vi "FlexMag - 23-03-2023.vi"() -> ()   [LabVIEW 2018] (continued)
            n880 = local read "CH3_CC_DI"() -> (w1149:bool)
            n881 = local read "Tp3_stop_cmnd"() -> (w1127:bool)
            n882 = local read "CH3_BG_BV_DI"() -> (w1124:bool)
            n883 = local read "CH3_TP_BV_DI"() -> (w1122:bool)
            n884 = Compound Arithmetic op=AND(w1091, w1092) -> (w1095:bool)
            n885 = Compound Arithmetic op=AND(w1093, w1094) -> (w1096:bool)
            n886 = local read "Tp3 speed gui"() -> (w1121:i32)
            n887 = local read "CH3_CC_DI"() -> (w1123:bool)
            n888 = local read "CH3_SoV_Ar_DI"() -> (w1141:bool)
            n889 = Or(x=w1095, y=w1096) -> (x .or. y?=w1086:bool)
            n890 = Not(x=w1149) -> (.not. x?=w1148:bool)
            n891 = Not(x=w1147) -> (.not. x?=w1146:bool)
            n892 = Not(x=w1145) -> (.not. x?=w1144:bool)
            n893 = local write "ch3 trnsbp right open safety"(w1086) -> ()
            n894 = Less Or Equal?(x=w1121, y=180) -> (x <= y?=w1119:bool)
            n895 = Not(x=w1124) -> (.not. x?=w1125:bool)
            n896 = Not(x=w1123) -> (.not. x?=w1126:bool)
            n897 = Not(x=w1122) -> (.not. x?=w1120:bool)
            n898 = Compound Arithmetic op=AND(w1148, w1146, w1144) -> (w1142:bool)
            n899 = Compound Arithmetic op=AND(w1127, w1125, w1126, w1120, w1119, w1117) -> (w1118:bool)
            n900 = local write "sov3 open safety"(w1142) -> ()
            n901 = Compound Arithmetic op=AND(w1142, w1141) -> (w1143:bool)
            n902 = local write "chvbv3 open safety"(w1118) -> ()
            n903 = local write "ch3 mfc set safety"(w1143) -> ()
          }
          frame True {
            w1166 = TRUE ("bgbv3 open safety")
            n904 = local write "bgbv3 open safety"(w1166) -> ()
            n905 = local write "cc3 open safety"(w1166) -> ()
            n906 = local write "tpbv3 open safety"(w1166) -> ()
            n907 = local write "mp3 stop safety"(w1166) -> ()
            n908 = local write "tp3 start safety"(w1166) -> ()
            n909 = local write "tpbv3 close safety"(w1166) -> ()
            n910 = local write "mp3 start safety"(w1166) -> ()
            n911 = local write "plvbv3 open safety"(w1166) -> ()
            n912 = local write "sov3 open safety"(w1166) -> ()
            n913 = local write "ch3 mfc set safety"(w1166) -> ()
            n914 = local write "chvbv3 open safety"(w1166) -> ()
            n915 = local write "ch3 trnsbp left open safety"(w1166) -> ()
            n916 = local write "ch3 trnsbp right open safety"(w1166) -> ()
          }
        }
        n917 = case shown="False" "CH4 safety cancel" {
          frame False {
            n918 = local read "CH4_CH_VBV_DI"() -> (w1069:bool)
            n919 = local read "CH4_PL_VBV_DI"() -> (w1030:bool)
            n920 = local read "CH4_PL_ATM_DI"() -> (w997:bool)
            n921 = local read "CH3_SoV_Ar_DI"() -> (w1066:bool)
            n922 = local read "CH4_CH_ATM_DI"() -> (w996:bool)
            n923 = local read "ch4 ch pg torr"() -> (w1072:dbl)
            n924 = local read "Tp4_stop_cmnd"() -> (w1002:bool)
            n925 = local read "CH4_TP_BV_DI"() -> (w1017:bool)
            n926 = local read "CH4_MP_DI"() -> (w1026:bool)
            n927 = local read "ch3_4 vacuum level"() -> (w1014:string)
            n928 = local read "ch4 ch pg torr"() -> (w1012:dbl)
            n929 = local read "ch4 ch pg torr"() -> (w1011:dbl)
            n930 = Not(x=w1030) -> (.not. x?=w1029:bool)
            n931 = Not(x=w1069) -> (.not. x?=w1068:bool)
            n932 = Less Or Equal?(x=w1072, y=0.09) -> (x <= y?=w1070:bool)
            n933 = Not(x=w1066) -> (.not. x?=w1067:bool)
            n934 = Not(x=w1017) -> (.not. x?=w1018:bool)
            n935 = Compound Arithmetic op=XOR(w997, w996) -> (w999:bool)
            n936 = Compound Arithmetic op=AND(w1026, w1068, w1070) -> (w1065:bool)
            n937 = Not(x=w999) -> (.not. x?=w998:bool)
            n938 = Compound Arithmetic op=AND(w1018, w1002) -> (w1019:bool)
            n939 = Greater Or Equal?(x=w1012, y=0.9) -> (x >= y?=w1010:bool)
            n940 = Equal?(x="ATMOSPHERE" ("y"), y=w1014) -> (x = y?=w1009:bool)
            n941 = Equal?(x=w1014, y="VACUUM") -> (x = y?=w1007:bool)
            n942 = Less Or Equal?(x=w1011, y=0.1) -> (x <= y?=w1006:bool)
            n943 = Compound Arithmetic op=AND(w1065, w1067) -> (w1064:bool)
            n944 = local write "bgbv4 open safety"(w1065) -> ()
            n945 = Compound Arithmetic op=AND(w998, w1029) -> (w1031:bool)
            n946 = local write "mp4 stop safety"(w1019) -> ()
            n947 = local write "cc4 open safety"(w1064) -> ()
            n948 = Compound Arithmetic op=AND(w1010, w1009) -> (w1005:bool)
            n949 = Compound Arithmetic op=AND(w1007, w1006) -> (w1004:bool)
            n950 = local write "tpbv4 open safety"(w1031) -> ()
            n951 = Or(x=w1005, y=w1004) -> (x .or. y?=w1003:bool)
            n952 = local write "ch4 trnsbp right open safety"(w1003) -> ()
            n953 = local read "CH4_CH_VBV_DI"() -> (w1062:bool)
            n954 = local read "Tp4_stop_cmnd"() -> (w1027:bool)
            n955 = local read "CH4_TP_BV_DI"() -> (w1058:bool)
            n956 = local read "ch4 ch pg torr"() -> (w1059:dbl)
            n957 = local read "CH4_TP_BV_DI"() -> (w1045:bool)
            n958 = local read "CH4_CH_VBV_DI"() -> (w1023:bool)
            n959 = local read "CH4_MP_DI"() -> (w1057:bool)
            n960 = local read "CH4_PL_VBV_DI"() -> (w1024:bool)
            n961 = local read "ch4_tp_gui"() -> (w1001:bool)
            n962 = local read "CH4_MP_DI"() -> (w1046:bool)
            n963 = Not(x=w1062) -> (.not. x?=w1063:bool)
            n964 = Less Or Equal?(x=w1059, y=0.7) -> (x <= y?=w1061:bool)
            n965 = Not(x=w1001) -> (.not. x?=w1000:bool)
            n966 = Not(x=w1045) -> (.not. x?=w1044:bool)
            n967 = Not(x=w1046) -> (.not. x?=w1043:bool)
            n968 = Not(x=w1023) -> (.not. x?=w1021:bool)
            n969 = Not(x=w1024) -> (.not. x?=w1022:bool)
            n970 = Compound Arithmetic op=AND(w1063, w1061, w1058, w1057) -> (w1056:bool)
            n971 = Compound Arithmetic op=AND(w1000, w1027) -> (w1028:bool)
            n972 = Compound Arithmetic op=AND(w1044, w1043) -> (w1042:bool)
            n973 = Compound Arithmetic op=AND(w1022, w1021) -> (w1020:bool)
            n974 = local write "tp4 start safety"(w1056) -> ()
            n975 = local write "tpbv4 close safety"(w1028) -> ()
            n976 = local write "mp4 start safety"(w1020) -> ()
            n977 = local write "plvbv4 open safety"(w1042) -> ()
            n978 = local read "CH4_CH_ATM_DI"() -> (w1054:bool)
            n979 = local read "CH4_CH_VBV_DI"() -> (w1052:bool)
            n980 = local read "Tp4_stop_cmnd"() -> (w1025:bool)
            n981 = local read "CH4_BG_BV_DI"() -> (w1039:bool)
            n982 = local read "CH4_TP_BV_DI"() -> (w1037:bool)
            n983 = local read "CH4_CC_DI"() -> (w1050:bool)
            n984 = local read "Tp4 speed gui"() -> (w1036:i32)
            n985 = local read "CH4_CC_DI"() -> (w1038:bool)
            n986 = local read "CH4_SoV_Ar_DI"() -> (w1048:bool)
            n987 = Not(x=w1050) -> (.not. x?=w1051:bool)
            n988 = Not(x=w1052) -> (.not. x?=w1053:bool)
            n989 = Not(x=w1054) -> (.not. x?=w1055:bool)
            n990 = Less Or Equal?(x=w1036, y=180) -> (x <= y?=w1033:bool)
            n991 = Not(x=w1039) -> (.not. x?=w1040:bool)
            n992 = Not(x=w1038) -> (.not. x?=w1041:bool)
            n993 = Not(x=w1037) -> (.not. x?=w1034:bool)
            n994 = Compound Arithmetic op=AND(w1025, w1040, w1041, w1034, w1033) -> (w1032:bool)
            n995 = Compound Arithmetic op=AND(w1051, w1053, w1055) -> (w1047:bool)
            n996 = Compound Arithmetic op=AND(w1047, w1048) -> (w1049:bool)
            n997 = local write "sov4 open safety"(w1047) -> ()
            n998 = local write "chvbv4 open safety"(w1032) -> ()
            n999 = local write "ch4 mfc set safety"(w1049) -> ()
          }
          frame True {
            w1073 = TRUE ("bgbv3 open safety")
            n1000 = local write "bgbv4 open safety"(w1073) -> ()
            n1001 = local write "cc4 open safety"(w1073) -> ()
            n1002 = local write "tpbv4 open safety"(w1073) -> ()
            n1003 = local write "mp4 stop safety"(w1073) -> ()
            n1004 = local write "tp4 start safety"(w1073) -> ()
            n1005 = local write "tpbv4 close safety"(w1073) -> ()
            n1006 = local write "mp4 start safety"(w1073) -> ()
            n1007 = local write "plvbv4 open safety"(w1073) -> ()
            n1008 = local write "sov4 open safety"(w1073) -> ()
            n1009 = local write "ch4 mfc set safety"(w1073) -> ()
            n1010 = local write "chvbv4 open safety"(w1073) -> ()
            n1011 = local write "ch4 trnsbp right open safety"(w1073) -> ()
          }
        }
        n1012 = case shown="False" "coating safety cancel" {
          frame False {
            n1013 = local read "ch2 argon mfc actual"() -> (w941:dbl)
            n1014 = local read "ch3 argon mfc actual"() -> (w944:dbl)
            n1015 = local read "CH2_SoV_Ar_DI"() -> (w946:bool)
            n1016 = local read "CH3_SoV_Ar_DI"() -> (w945:bool)
            n1017 = local read "DCPS_ SW1 DI"() -> (w952:bool)
            n1018 = local read "DCPS_ SW2 DI"() -> (w950:bool)
            n1019 = local read "CH2_WFC_DI"() -> (w951:bool)
            n1020 = local read "CH3_WFC_DI"() -> (w949:bool)
            n1021 = Greater Or Equal?(x=w941, y=3.0) -> (x >= y?=w940:bool)
            n1022 = Greater Or Equal?(x=w944, y=3.0) -> (x >= y?=w939:bool)
            n1023 = Compound Arithmetic op=AND(w940, w946, w952, w951) -> (w948:bool)
            n1024 = Compound Arithmetic op=AND(w949, w950, w945, w939) -> (w947:bool)
            n1025 = Or(x=w948, y=w947) -> (x .or. y?=w938:bool)
            n1026 = local write "dcps on safety"(w938) -> ()
          }
          frame True {
            n1027 = local write "dcps on safety"(TRUE ("dcps on safety")) -> ()
          }
        }
        n1028 = case shown="False" "trns safety cancel" {
          frame False {
            n1029 = local read "ch1 ch pg torr"() -> (w992:dbl)
            n1030 = local read "ch2 ch pg torr"() -> (w987:dbl)
            n1031 = local read "ch2 ch pg torr"() -> (w969:dbl)
            n1032 = local read "ch3 ch pg torr"() -> (w974:dbl)
            n1033 = local read "ch3 ch pg torr"() -> (w968:dbl)
            n1034 = local read "ch4 ch pg torr"() -> (w963:dbl)
            n1035 = local read "Casette_Servo_Start/Stop DI"() -> (w994:bool)
            n1036 = Greater Or Equal?(x=w992, y=0.9) -> (x >= y?=w986:bool)
            n1037 = Less?(x=w992, y=0.1) -> (x < y?=w983:bool)
            n1038 = Greater Or Equal?(x=w987, y=0.9) -> (x >= y?=w985:bool)
            n1039 = Less?(x=w987, y=0.1) -> (x < y?=w984:bool)
            n1040 = Greater Or Equal?(x=w969, y=0.9) -> (x >= y?=w975:bool)
            n1041 = Less?(x=w969, y=0.1) -> (x < y?=w978:bool)
            n1042 = Greater Or Equal?(x=w974, y=0.9) -> (x >= y?=w976:bool)
            n1043 = Less?(x=w974, y=0.1) -> (x < y?=w977:bool)
            n1044 = Greater Or Equal?(x=w968, y=0.9) -> (x >= y?=w962:bool)
            n1045 = Less?(x=w968, y=0.1) -> (x < y?=w959:bool)
            n1046 = Greater Or Equal?(x=w963, y=0.9) -> (x >= y?=w961:bool)
            n1047 = Less?(x=w963, y=0.1) -> (x < y?=w960:bool)
            n1048 = Not(x=w994) -> (.not. x?=w993:bool)
            n1049 = local write "CH1-2 trns close safety"(w993) -> ()
            n1050 = local write "CH2-3 trns close safety"(w993) -> ()
            n1051 = local write "CH3-4 trns close safety"(w993) -> ()
            n1052 = Compound Arithmetic op=AND(w986, w985) -> (w982:bool)
            n1053 = Compound Arithmetic op=AND(w983, w984) -> (w981:bool)
            n1054 = Compound Arithmetic op=AND(w975, w976) -> (w979:bool)
            n1055 = Compound Arithmetic op=AND(w978, w977) -> (w980:bool)
            n1056 = Compound Arithmetic op=AND(w962, w961) -> (w958:bool)
            n1057 = Compound Arithmetic op=AND(w959, w960) -> (w957:bool)
            n1058 = Compound Arithmetic op=OR(w982, w981) -> (w956:bool)
            n1059 = Compound Arithmetic op=OR(w979, w980) -> (w955:bool)
            n1060 = Compound Arithmetic op=OR(w958, w957) -> (w954:bool)
            n1061 = local write "CH2-3 trns open safety"(w955) -> ()
            n1062 = local write "CH3-4 trns open safety"(w954) -> ()
            n1063 = local write "CH1-2 trns open safety"(w956) -> ()
          }
          frame True {
            w995 = TRUE
            n1064 = local write "CH1-2 trns close safety"(w995) -> ()
            n1065 = local write "CH2-3 trns close safety"(w995) -> ()
            n1066 = local write "CH3-4 trns close safety"(w995) -> ()
            n1067 = local write "CH1-2 trns open safety"(w995) -> ()
            n1068 = local write "CH2-3 trns open safety"(w995) -> ()
            n1069 = local write "CH3-4 trns open safety"(w995) -> ()
          }
        }
      }
    }
    n1070 = Wait Until Next ms Multiple(millisecond multiple=u32 300) -> ()  [unwired: 1 out]
  }
  n1071 = while {
    stop <- FALSE stop-if-true
    n1072 = stacked-sequence {
      frame #0 {
        n1073 = local read "DCPS_ SW1 DI"() -> (w1346:bool)
        "CH2 MAG Active" <- w1346
        n1074 = local read "DCPS_ SW2 DI"() -> (w1349:bool)
        "CH3 MAG Active" <- w1349
        n1075 = case shown="True" "CH2 water close gui" {
          frame False {
          }
          frame True {
            n1076 = local write "CH2_WFC_DO"(FALSE ("CH2_WFC_DO")) -> ()
            n1077 = Wait (ms)(milliseconds to wait=u32 100) -> ()  [unwired: 1 out]
          }
        }
        n1078 = case shown="True" "CH2 water open gui" {
          frame False {
          }
          frame True {
            n1079 = local write "CH1_WFC_DO"(FALSE ("CH1_WFC_DO")) -> ()
            n1080 = local write "CH2_WFC_DO"(TRUE ("CH2_WFC_DO")) -> ()
            n1081 = local write "CH3_WFC_DO"(FALSE ("CH3_WFC_DO")) -> ()
            n1082 = local write "CH4_WFC_DO"(FALSE ("CH4_WFC_DO")) -> ()
            n1083 = Wait (ms)(milliseconds to wait=u32 100) -> ()  [unwired: 1 out]
          }
        }
        n1084 = Or(x=w1346, y=w1349) -> (x .or. y?=w1348:bool)
        n1085 = case shown="True" w1348 {
          tunnel: [FALSE TRUE] -> w1347
          tunnel: w1346 -> [_ w1367]
          tunnel: [FALSE ("DCPS_ SW1 DI") w1367] -> w1345
          frame False {
          }
          frame True {
          }
        }
        "MAG gui" <- w1345
        n1086 = property on="MAG gui" class="Bool (strict)"("Visible"=w1347) -> ()  [unwired: 2 in, 2 out]
        n1087 = case shown="True" "CH3 water close gui" {
          frame False {
          }
          frame True {
            n1088 = local write "CH3_WFC_DO"(FALSE ("CH2_WFC_DO")) -> ()
            n1089 = Wait (ms)(milliseconds to wait=u32 100) -> ()  [unwired: 1 out]
          }
        }
        n1090 = case shown="True" "CH3 water open gui" {
          frame False {
          }
          frame True {
            n1091 = local write "CH1_WFC_DO"(FALSE ("CH1_WFC_DO")) -> ()
            n1092 = local write "CH2_WFC_DO"(FALSE ("CH2_WFC_DO")) -> ()
            n1093 = local write "CH3_WFC_DO"(TRUE ("CH3_WFC_DO")) -> ()
            n1094 = local write "CH4_WFC_DO"(FALSE ("CH4_WFC_DO")) -> ()
            n1095 = Wait (ms)(milliseconds to wait=u32 100) -> ()  [unwired: 1 out]
          }
        }
      }
      frame #1 {
        n1096 = local read "CH1_SRV1_Piston_Back_DO"() -> (w1407:bool)
        n1097 = local read "CH1_SRV1_Piston_Back_DI"() -> (w1408:bool)
        n1098 = local read "CH1_SRV1_Piston_For_DO"() -> (w1390:bool)
        n1099 = local read "CH1_SRV1_Piston_For_DI"() -> (w1389:bool)
        n1100 = local read "CH1_CH_VBV_DO"() -> (w1449:bool)
        n1101 = local read "CH1_CH_VBV_DI"() -> (w1448:bool)
        n1102 = local read "CH1_SRV_Start_Stop_DI"() -> (w1368:bool)
        n1103 = local read "CH1_MP_DO"() -> (w1459:bool)
        n1104 = local read "CH1_MP_DI"() -> (w1458:bool)
        n1105 = local read "CH1_TP_BV_DO"() -> (w1456:bool)
        n1106 = local read "CH1_TP_BV_DI"() -> (w1457:bool)
        n1107 = local read "CH1_BG_BV_DO"() -> (w1446:bool)
        n1108 = local read "CH1_BG_BV_DI"() -> (w1447:bool)
        n1109 = local read "CH1_M3_D3_DO"() -> (w1369:bool)
        n1110 = local read "CH1_Cst_Fix_Down_DI"() -> (w1409:bool)
        n1111 = local read "CH1_WFC_DO"() -> (w1387:bool)
        n1112 = local read "CH1_WFC_DI"() -> (w1388:bool)
        n1113 = local read "CH1_Cst_Fix_DO"() -> (w1410:bool)
        n1114 = feedback #1() -> (w1444:bool)  [unwired: 1 in]
        n1115 = Exclusive Or(1:w1447, 2:w1446) -> (0:w1443:bool)
        n1116 = feedback #2() -> (w1451:bool)  [unwired: 1 in]
        n1117 = Exclusive Or(1:w1448, 2:w1449) -> (0:w1452:bool)
        n1118 = feedback #3() -> (w1461:bool)  [unwired: 1 in]
        n1119 = Exclusive Or(1:w1458, 2:w1459) -> (0:w1462:bool)
        n1120 = feedback #4() -> (w1454:bool)  [unwired: 1 in]
        n1121 = Exclusive Or(1:w1457, 2:w1456) -> (0:w1453:bool)
        n1122 = feedback #5() -> (w1371:bool)  [unwired: 1 in]
        n1123 = Exclusive Or(1:w1368, 2:w1369) -> (0:w1372:bool)
        n1124 = case shown="True" w1443 {
          tunnel: w1444 -> [_ w1563]
          tunnel: [TRUE FALSE] -> w1445
          tunnel: [FALSE w1564] -> w1423
          frame False {
          }
          frame True {
            n1125 = call "Elapsed Time79"("Reset"=w1563) -> ("Elapsed Time (s)"=w1565:dbl)  [unwired: 11 in, 7 out]
            n1126 = Greater Or Equal?(x=w1565, y=5.0) -> (x >= y?=w1564:bool)
          }
        }
        n1127 = feedback-in #1(w1445) -> ()
        n1128 = case shown="True" w1452 {
          tunnel: w1451 -> [_ w1556]
          tunnel: [TRUE FALSE] -> w1450
          tunnel: [FALSE w1557] -> w1425
          frame False {
          }
          frame True {
            n1129 = call "Elapsed Time80"("Reset"=w1556) -> ("Elapsed Time (s)"=w1558:dbl)  [unwired: 11 in, 7 out]
            n1130 = Greater Or Equal?(x=w1558, y=5.0) -> (x >= y?=w1557:bool)
          }
        }
        n1131 = feedback-in #2(w1450) -> ()
        n1132 = feedback #6() -> (w1385:bool)  [unwired: 1 in]
        n1133 = Exclusive Or(1:w1388, 2:w1387) -> (0:w1384:bool)
        n1134 = case shown="True" w1462 {
          tunnel: w1461 -> [_ w1577]
          tunnel: [TRUE FALSE] -> w1460
          tunnel: [FALSE w1578] -> w1427
          frame False {
          }
          frame True {
            n1135 = call "Elapsed Time77"("Reset"=w1577) -> ("Elapsed Time (s)"=w1579:dbl)  [unwired: 11 in, 7 out]
            n1136 = Greater Or Equal?(x=w1579, y=5.0) -> (x >= y?=w1578:bool)
          }
        }
        n1137 = feedback-in #3(w1460) -> ()
        n1138 = case shown="True" w1453 {
          tunnel: w1454 -> [_ w1570]
          tunnel: [TRUE FALSE] -> w1455
          tunnel: [FALSE w1571] -> w1424
          frame False {
          }
          frame True {
            n1139 = call "Elapsed Time78"("Reset"=w1570) -> ("Elapsed Time (s)"=w1572:dbl)  [unwired: 11 in, 7 out]
            n1140 = Greater Or Equal?(x=w1572, y=5.0) -> (x >= y?=w1571:bool)
          }
        }
        n1141 = feedback-in #4(w1455) -> ()
        n1142 = feedback #7() -> (w1412:bool)  [unwired: 1 in]
        n1143 = Exclusive Or(1:w1409, 2:w1410) -> (0:w1413:bool)
        n1144 = feedback #8() -> (w1405:bool)  [unwired: 1 in]
        n1145 = Exclusive Or(1:w1408, 2:w1407) -> (0:w1404:bool)
        n1146 = feedback #9() -> (w1392:bool)  [unwired: 1 in]
        n1147 = Exclusive Or(1:w1389, 2:w1390) -> (0:w1393:bool)
        n1148 = case shown="True" w1372 {
          tunnel: w1371 -> [_ w1465]
          tunnel: [TRUE FALSE] -> w1370
          tunnel: [FALSE w1466] -> _
          frame False {
          }
          frame True {
            n1149 = call "Elapsed Time82"("Reset"=w1465) -> ("Elapsed Time (s)"=w1467:dbl)  [unwired: 11 in, 7 out]
            n1150 = Greater Or Equal?(x=w1467, y=5.0) -> (x >= y?=w1466:bool)
          }
        }
        n1151 = feedback-in #5(w1370) -> ()
        n1152 = case shown="True" w1384 {
          tunnel: w1385 -> [_ w1486]
          tunnel: [TRUE FALSE] -> w1386
          tunnel: [FALSE w1487] -> _
          frame False {
          }
          frame True {
            n1153 = call "Elapsed Time93"("Reset"=w1486) -> ("Elapsed Time (s)"=w1488:dbl)  [unwired: 11 in, 7 out]
            n1154 = Greater Or Equal?(x=w1488, y=5.0) -> (x >= y?=w1487:bool)
          }
        }
        n1155 = feedback-in #6(w1386) -> ()
        n1156 = case shown="True" w1413 {
          tunnel: w1412 -> [_ w1521]
          tunnel: [TRUE FALSE] -> w1411
          tunnel: [FALSE w1522] -> _
          frame False {
          }
          frame True {
            n1157 = call "Elapsed Time88"("Reset"=w1521) -> ("Elapsed Time (s)"=w1523:dbl)  [unwired: 11 in, 7 out]
            n1158 = Greater Or Equal?(x=w1523, y=20.0) -> (x >= y?=w1522:bool)
          }
        }
        n1159 = feedback-in #7(w1411) -> ()
        n1160 = case shown="True" w1404 {
          tunnel: w1405 -> [_ w1514]
          tunnel: [TRUE FALSE] -> w1406
          tunnel: [FALSE w1515] -> _
          frame False {
          }
          frame True {
            n1161 = call "Elapsed Time89"("Reset"=w1514) -> ("Elapsed Time (s)"=w1516:dbl)  [unwired: 11 in, 7 out]
            n1162 = Greater Or Equal?(x=w1516, y=25.0) -> (x >= y?=w1515:bool)
          }
        }
        n1163 = feedback-in #8(w1406) -> ()
        n1164 = case shown="True" w1393 {
          tunnel: w1392 -> [_ w1493]
          tunnel: [TRUE FALSE] -> w1391
          tunnel: [FALSE w1494] -> _
          frame False {
          }
          frame True {
            n1165 = call "Elapsed Time92"("Reset"=w1493) -> ("Elapsed Time (s)"=w1495:dbl)  [unwired: 11 in, 7 out]
            n1166 = Greater Or Equal?(x=w1495, y=25.0) -> (x >= y?=w1494:bool)
          }
        }
        n1167 = feedback-in #9(w1391) -> ()
        n1168 = local write "ch1_ch_vbv_fail"(w1425) -> ()
        n1169 = local write "ch1_mp_fail"(w1427) -> ()
        n1170 = local write "ch1_tp_bv_fail"(w1424) -> ()
        n1171 = local write "ch1_bg_bv_fail"(w1423) -> ()
        n1172 = local read "CH1_PetCool_Down_DO"() -> (w1400:bool)
        n1173 = local read "CH1_PetCool_Down_DI"() -> (w1399:bool)
        n1174 = local read "CH1_Trns_Gv_Open_DO"() -> (w1436:bool)
        n1175 = local read "CH1_Trns_Gv_Open_DI"() -> (w1437:bool)
        n1176 = local read "CH1_Trns_Gv_Close_DO"() -> (w1419:bool)
        n1177 = local read "CH1_Trns_Gv_Close_DI"() -> (w1418:bool)
        n1178 = local read "CH1_Trns_BP_Left_DO"() -> (w1380:bool)
        n1179 = local read "CH1_Trns_BP_Left_DI"() -> (w1379:bool)
        n1180 = local read "CH1_TGV_Control_DO"() -> (w1376:bool)
        n1181 = local read "CH1_TGV_Control_DI"() -> (w1377:bool)
        n1182 = local read "CH1_PetCool_Up_DO"() -> (w1397:bool)
        n1183 = local read "CH1_PetCool_Up_DI"() -> (w1398:bool)
        n1184 = local read "CH1_PL_VBV_DO"() -> (w1431:bool)
        n1185 = local read "CH1_PL_VBV_DI"() -> (w1432:bool)
        n1186 = local read "CH1_SoV_Ar_DO"() -> (w1439:bool)
        n1187 = local read "CH1_SoV_Ar_DI"() -> (w1438:bool)
        n1188 = feedback #10() -> (w1429:bool)  [unwired: 1 in]
        n1189 = Exclusive Or(1:w1432, 2:w1431) -> (0:w1428:bool)
        n1190 = feedback #11() -> (w1441:bool)  [unwired: 1 in]
        n1191 = Exclusive Or(1:w1438, 2:w1439) -> (0:w1442:bool)
        n1192 = feedback #12() -> (w1434:bool)  [unwired: 1 in]
        n1193 = Exclusive Or(1:w1437, 2:w1436) -> (0:w1433:bool)
        n1194 = feedback #13() -> (w1421:bool)  [unwired: 1 in]
        n1195 = Exclusive Or(1:w1418, 2:w1419) -> (0:w1422:bool)
        n1196 = feedback #14() -> (w1395:bool)  [unwired: 1 in]
        n1197 = Exclusive Or(1:w1398, 2:w1397) -> (0:w1394:bool)
        n1198 = feedback #15() -> (w1402:bool)  [unwired: 1 in]
        n1199 = Exclusive Or(1:w1399, 2:w1400) -> (0:w1403:bool)
        n1200 = feedback #16() -> (w1382:bool)  [unwired: 1 in]
        n1201 = Exclusive Or(1:w1379, 2:w1380) -> (0:w1383:bool)
        n1202 = feedback #17() -> (w1374:bool)  [unwired: 1 in]
        n1203 = Exclusive Or(1:w1377, 2:w1376) -> (0:w1373:bool)
        n1204 = case shown="True" w1428 {
          tunnel: w1429 -> [_ w1549]
          tunnel: [TRUE FALSE] -> w1430
          tunnel: [FALSE w1550] -> w1426
          frame False {
          }
          frame True {
            n1205 = call "Elapsed Time81"("Reset"=w1549) -> ("Elapsed Time (s)"=w1551:dbl)  [unwired: 11 in, 7 out]
            n1206 = Greater Or Equal?(x=w1551, y=5.0) -> (x >= y?=w1550:bool)
          }
        }
        n1207 = feedback-in #10(w1430) -> ()
        n1208 = case shown="True" w1442 {
          tunnel: w1441 -> [_ w1542]
          tunnel: [TRUE FALSE] -> w1440
          tunnel: [FALSE w1543] -> w1414
          frame False {
          }
          frame True {
            n1209 = call "Elapsed Time83"("Reset"=w1542) -> ("Elapsed Time (s)"=w1544:dbl)  [unwired: 11 in, 7 out]
            n1210 = Greater Or Equal?(x=w1544, y=5.0) -> (x >= y?=w1543:bool)
          }
        }
        n1211 = feedback-in #11(w1440) -> ()
        n1212 = case shown="True" w1433 {
          tunnel: w1434 -> [_ w1535]
          tunnel: [TRUE FALSE] -> w1435
          tunnel: [FALSE w1536] -> w1416
          frame False {
          }
          frame True {
            n1213 = call "Elapsed Time84"("Reset"=w1535) -> ("Elapsed Time (s)"=w1537:dbl)  [unwired: 11 in, 7 out]
            n1214 = Greater Or Equal?(x=w1537, y=30.0) -> (x >= y?=w1536:bool)
          }
        }
        n1215 = feedback-in #12(w1435) -> ()
        n1216 = case shown="True" w1422 {
          tunnel: w1421 -> [_ w1528]
          tunnel: [TRUE FALSE] -> w1420
          tunnel: [FALSE w1529] -> w1415
          frame False {
          }
          frame True {
            n1217 = call "Elapsed Time70"("Reset"=w1528) -> ("Elapsed Time (s)"=w1530:dbl)  [unwired: 11 in, 7 out]
            n1218 = Greater Or Equal?(x=w1530, y=30.0) -> (x >= y?=w1529:bool)
          }
        }
        n1219 = feedback-in #13(w1420) -> ()
        n1220 = case shown="True" w1394 {
          tunnel: w1395 -> [_ w1507]
          tunnel: [TRUE FALSE] -> w1396
          tunnel: [FALSE w1508] -> _
          frame False {
          }
          frame True {
            n1221 = call "Elapsed Time90"("Reset"=w1507) -> ("Elapsed Time (s)"=w1509:dbl)  [unwired: 11 in, 7 out]
            n1222 = Greater Or Equal?(x=w1509, y=25.0) -> (x >= y?=w1508:bool)
          }
        }
        n1223 = feedback-in #14(w1396) -> ()
        n1224 = case shown="True" w1403 {
          tunnel: w1402 -> [_ w1500]
          tunnel: [TRUE FALSE] -> w1401
          tunnel: [FALSE w1501] -> _
          frame False {
          }
          frame True {
            n1225 = call "Elapsed Time91"("Reset"=w1500) -> ("Elapsed Time (s)"=w1502:dbl)  [unwired: 11 in, 7 out]
            n1226 = Greater Or Equal?(x=w1502, y=25.0) -> (x >= y?=w1501:bool)
          }
        }
        n1227 = feedback-in #15(w1401) -> ()
        n1228 = case shown="True" w1383 {
          tunnel: w1382 -> [_ w1479]
          tunnel: [TRUE FALSE] -> w1381
          tunnel: [FALSE w1480] -> w1378
          frame False {
          }
          frame True {
            n1229 = call "Elapsed Time94"("Reset"=w1479) -> ("Elapsed Time (s)"=w1481:dbl)  [unwired: 11 in, 7 out]
            n1230 = Greater Or Equal?(x=w1481, y=10.0) -> (x >= y?=w1480:bool)
          }
        }
        n1231 = feedback-in #16(w1381) -> ()
        n1232 = case shown="True" w1373 {
          tunnel: w1374 -> [_ w1472]
          tunnel: [TRUE FALSE] -> w1375
          tunnel: [FALSE w1473] -> _
          frame False {
          }
          frame True {
            n1233 = call "Elapsed Time95"("Reset"=w1472) -> ("Elapsed Time (s)"=w1474:dbl)  [unwired: 11 in, 7 out]
            n1234 = Greater Or Equal?(x=w1474, y=5.0) -> (x >= y?=w1473:bool)
          }
        }
        n1235 = feedback-in #17(w1375) -> ()
        n1236 = local write "ch1_pl_vbv_fail"(w1426) -> ()
        n1237 = local write "ch1_sov_fail"(w1414) -> ()
        n1238 = Or(x=w1416, y=w1415) -> (x .or. y?=w1417:bool)
        n1239 = local write "ch1_gv_bp_left_fail"(w1378) -> ()
        n1240 = local write "ch1_2_trns_gv_fail"(w1417) -> ()
      }
      frame #2 {
        n1241 = local read "CH2_SRV1_Piston_Back_DO"() -> (w1627:bool)
        n1242 = local read "CH2_SRV1_Piston_Back_DI"() -> (w1628:bool)
        n1243 = local read "CH2_SRV1_Piston_For_DO"() -> (w1610:bool)
        n1244 = local read "CH2_SRV1_Piston_For_DI"() -> (w1609:bool)
        n1245 = local read "CH2_CH_VBV_DO"() -> (w1669:bool)
        n1246 = local read "CH2_CH_VBV_DI"() -> (w1668:bool)
        n1247 = local read "CH2_SRV_Start_Stop_DI"() -> (w1588:bool)
        n1248 = local read "CH2_MP_DO"() -> (w1679:bool)
        n1249 = local read "CH2_MP_DI"() -> (w1678:bool)
        n1250 = local read "CH2_TP_BV_DO"() -> (w1676:bool)
        n1251 = local read "CH2_TP_BV_DI"() -> (w1677:bool)
        n1252 = local read "CH2_BG_BV_DO"() -> (w1666:bool)
        n1253 = local read "CH2_BG_BV_DI"() -> (w1667:bool)
        n1254 = local read "CH2_M3_D3_DO"() -> (w1589:bool)
        n1255 = local read "CH2_Cst_Fix_Down_DI"() -> (w1629:bool)
        n1256 = local read "CH2_WFC_DO"() -> (w1607:bool)
        n1257 = local read "CH2_WFC_DI"() -> (w1608:bool)
        n1258 = local read "CH2_Cst_Fix_DO"() -> (w1630:bool)
        n1259 = feedback #18() -> (w1664:bool)  [unwired: 1 in]
        n1260 = Exclusive Or(1:w1667, 2:w1666) -> (0:w1663:bool)
        n1261 = feedback #19() -> (w1671:bool)  [unwired: 1 in]
        n1262 = Exclusive Or(1:w1668, 2:w1669) -> (0:w1672:bool)
        n1263 = feedback #20() -> (w1681:bool)  [unwired: 1 in]
        n1264 = Exclusive Or(1:w1678, 2:w1679) -> (0:w1682:bool)
        n1265 = feedback #21() -> (w1674:bool)  [unwired: 1 in]
        n1266 = Exclusive Or(1:w1677, 2:w1676) -> (0:w1673:bool)
        n1267 = case shown="True" w1663 {
          tunnel: w1664 -> [_ w1790]
          tunnel: [TRUE FALSE] -> w1665
          tunnel: [FALSE w1791] -> w1643
          frame False {
          }
          frame True {
            n1268 = call "Elapsed Time98"("Reset"=w1790) -> ("Elapsed Time (s)"=w1792:dbl)  [unwired: 11 in, 7 out]
            n1269 = Greater Or Equal?(x=w1792, y=5.0) -> (x >= y?=w1791:bool)
          }
        }
        n1270 = feedback-in #18(w1665) -> ()
        n1271 = case shown="True" w1672 {
          tunnel: w1671 -> [_ w1783]
          tunnel: [TRUE FALSE] -> w1670
          tunnel: [FALSE w1784] -> w1645
          frame False {
          }
          frame True {
            n1272 = call "Elapsed Time99"("Reset"=w1783) -> ("Elapsed Time (s)"=w1785:dbl)  [unwired: 11 in, 7 out]
            n1273 = Greater Or Equal?(x=w1785, y=5.0) -> (x >= y?=w1784:bool)
          }
        }
        n1274 = feedback-in #19(w1670) -> ()
        n1275 = feedback #22() -> (w1605:bool)  [unwired: 1 in]
        n1276 = Exclusive Or(1:w1608, 2:w1607) -> (0:w1604:bool)
        n1277 = feedback #23() -> (w1591:bool)  [unwired: 1 in]
        n1278 = Exclusive Or(1:w1588, 2:w1589) -> (0:w1592:bool)
        n1279 = case shown="True" w1682 {
          tunnel: w1681 -> [_ w1804]
          tunnel: [TRUE FALSE] -> w1680
          tunnel: [FALSE w1805] -> w1647
          frame False {
          }
          frame True {
            n1280 = call "Elapsed Time96"("Reset"=w1804) -> ("Elapsed Time (s)"=w1806:dbl)  [unwired: 11 in, 7 out]
            n1281 = Greater Or Equal?(x=w1806, y=5.0) -> (x >= y?=w1805:bool)
          }
        }
        n1282 = feedback-in #20(w1680) -> ()
        n1283 = case shown="True" w1673 {
          tunnel: w1674 -> [_ w1797]
          tunnel: [TRUE FALSE] -> w1675
          tunnel: [FALSE w1798] -> w1644
          frame False {
          }
          frame True {
            n1284 = call "Elapsed Time97"("Reset"=w1797) -> ("Elapsed Time (s)"=w1799:dbl)  [unwired: 11 in, 7 out]
            n1285 = Greater Or Equal?(x=w1799, y=5.0) -> (x >= y?=w1798:bool)
          }
        }
        n1286 = feedback-in #21(w1675) -> ()
        n1287 = feedback #24() -> (w1632:bool)  [unwired: 1 in]
        n1288 = Exclusive Or(1:w1629, 2:w1630) -> (0:w1633:bool)
        n1289 = feedback #25() -> (w1625:bool)  [unwired: 1 in]
        n1290 = Exclusive Or(1:w1628, 2:w1627) -> (0:w1624:bool)
        n1291 = feedback #26() -> (w1612:bool)  [unwired: 1 in]
        n1292 = Exclusive Or(1:w1609, 2:w1610) -> (0:w1613:bool)
        n1293 = case shown="True" w1604 {
          tunnel: w1605 -> [_ w1713]
          tunnel: [TRUE FALSE] -> w1606
          tunnel: [FALSE w1714] -> _
          frame False {
          }
          frame True {
            n1294 = call "Elapsed Time110"("Reset"=w1713) -> ("Elapsed Time (s)"=w1715:dbl)  [unwired: 11 in, 7 out]
            n1295 = Greater Or Equal?(x=w1715, y=5.0) -> (x >= y?=w1714:bool)
          }
        }
        n1296 = feedback-in #22(w1606) -> ()
        n1297 = case shown="True" w1592 {
          tunnel: w1591 -> [_ w1692]
          tunnel: [TRUE FALSE] -> w1590
          tunnel: [FALSE w1693] -> _
          frame False {
          }
          frame True {
            n1298 = call "Elapsed Time101"("Reset"=w1692) -> ("Elapsed Time (s)"=w1694:dbl)  [unwired: 11 in, 7 out]
            n1299 = Greater Or Equal?(x=w1694, y=5.0) -> (x >= y?=w1693:bool)
          }
        }
        n1300 = feedback-in #23(w1590) -> ()
        n1301 = case shown="True" w1633 {
          tunnel: w1632 -> [_ w1748]
          tunnel: [TRUE FALSE] -> w1631
          tunnel: [FALSE w1749] -> _
          frame False {
          }
          frame True {
            n1302 = call "Elapsed Time105"("Reset"=w1748) -> ("Elapsed Time (s)"=w1750:dbl)  [unwired: 11 in, 7 out]
            n1303 = Greater Or Equal?(x=w1750, y=20.0) -> (x >= y?=w1749:bool)
          }
        }
        n1304 = feedback-in #24(w1631) -> ()
        n1305 = case shown="True" w1624 {
          tunnel: w1625 -> [_ w1741]
          tunnel: [TRUE FALSE] -> w1626
          tunnel: [FALSE w1742] -> _
          frame False {
          }
          frame True {
            n1306 = call "Elapsed Time106"("Reset"=w1741) -> ("Elapsed Time (s)"=w1743:dbl)  [unwired: 11 in, 7 out]
            n1307 = Greater Or Equal?(x=w1743, y=25.0) -> (x >= y?=w1742:bool)
          }
        }
        n1308 = feedback-in #25(w1626) -> ()
        n1309 = case shown="True" w1613 {
          tunnel: w1612 -> [_ w1720]
          tunnel: [TRUE FALSE] -> w1611
          tunnel: [FALSE w1721] -> _
          frame False {
          }
          frame True {
            n1310 = call "Elapsed Time109"("Reset"=w1720) -> ("Elapsed Time (s)"=w1722:dbl)  [unwired: 11 in, 7 out]
            n1311 = Greater Or Equal?(x=w1722, y=25.0) -> (x >= y?=w1721:bool)
          }
        }
        n1312 = feedback-in #26(w1611) -> ()
        n1313 = local write "ch2_ch_vbv_fail"(w1645) -> ()
        n1314 = local write "ch2_mp_fail"(w1647) -> ()
        n1315 = local write "ch2_tp_bv_fail"(w1644) -> ()
        n1316 = local write "ch2_bg_bv_fail"(w1643) -> ()
        n1317 = local read "CH2_PetCool_Down_DO"() -> (w1620:bool)
        n1318 = local read "CH2_PetCool_Down_DI"() -> (w1619:bool)
        n1319 = local read "CH2_Trns_GV_Open_DO"() -> (w1656:bool)
        n1320 = local read "CH2_Trns_GV_Close_DO"() -> (w1639:bool)
        n1321 = local read "CH2_Trns_BP_Right_DO"() -> (w1585:bool)
        n1322 = local read "CH2_Trns_BP_Right_DI"() -> (w1586:bool)
        n1323 = local read "CH2_Trns_Gv_Open_DI"() -> (w1657:bool)
        n1324 = local read "CH2_Trns_Gv_Close_DI"() -> (w1638:bool)
        n1325 = local read "CH2_Trns_BP_Left_DO"() -> (w1600:bool)
        n1326 = local read "CH2_Trns_BP_Left_DI"() -> (w1599:bool)
        n1327 = local read "CH2_TGV_Control_DO"() -> (w1596:bool)
        n1328 = local read "CH2_TGV_Control_DI"() -> (w1597:bool)
        n1329 = local read "CH2_PetCool_Up_DO"() -> (w1617:bool)
        n1330 = local read "CH2_PetCool_Up_DI"() -> (w1618:bool)
        n1331 = local read "CH2_PL_VBV_DO"() -> (w1651:bool)
        n1332 = local read "CH2_PL_VBV_DI"() -> (w1652:bool)
        n1333 = local read "CH2_SoV_Ar_DO"() -> (w1659:bool)
        n1334 = local read "CH2_SoV_Ar_DI"() -> (w1658:bool)
        n1335 = feedback #27() -> (w1649:bool)  [unwired: 1 in]
        n1336 = Exclusive Or(1:w1652, 2:w1651) -> (0:w1648:bool)
        n1337 = feedback #28() -> (w1661:bool)  [unwired: 1 in]
        n1338 = Exclusive Or(1:w1658, 2:w1659) -> (0:w1662:bool)
        n1339 = feedback #29() -> (w1654:bool)  [unwired: 1 in]
        n1340 = Exclusive Or(1:w1657, 2:w1656) -> (0:w1653:bool)
        n1341 = feedback #30() -> (w1641:bool)  [unwired: 1 in]
        n1342 = Exclusive Or(1:w1638, 2:w1639) -> (0:w1642:bool)
        n1343 = feedback #31() -> (w1615:bool)  [unwired: 1 in]
        n1344 = Exclusive Or(1:w1618, 2:w1617) -> (0:w1614:bool)
        n1345 = feedback #32() -> (w1622:bool)  [unwired: 1 in]
        n1346 = Exclusive Or(1:w1619, 2:w1620) -> (0:w1623:bool)
        n1347 = feedback #33() -> (w1602:bool)  [unwired: 1 in]
        n1348 = Exclusive Or(1:w1599, 2:w1600) -> (0:w1603:bool)
        n1349 = feedback #34() -> (w1583:bool)  [unwired: 1 in]
        n1350 = Exclusive Or(1:w1586, 2:w1585) -> (0:w1582:bool)
        n1351 = feedback #35() -> (w1594:bool)  [unwired: 1 in]
        n1352 = Exclusive Or(1:w1597, 2:w1596) -> (0:w1593:bool)
        n1353 = case shown="True" w1648 {
          tunnel: w1649 -> [_ w1776]
          tunnel: [TRUE FALSE] -> w1650
          tunnel: [FALSE w1777] -> w1646
          frame False {
          }
          frame True {
            n1354 = call "Elapsed Time100"("Reset"=w1776) -> ("Elapsed Time (s)"=w1778:dbl)  [unwired: 11 in, 7 out]
            n1355 = Greater Or Equal?(x=w1778, y=5.0) -> (x >= y?=w1777:bool)
          }
        }
        n1356 = feedback-in #27(w1650) -> ()
        n1357 = case shown="True" w1662 {
          tunnel: w1661 -> [_ w1769]
          tunnel: [TRUE FALSE] -> w1660
          tunnel: [FALSE w1770] -> w1634
          frame False {
          }
          frame True {
            n1358 = call "Elapsed Time102"("Reset"=w1769) -> ("Elapsed Time (s)"=w1771:dbl)  [unwired: 11 in, 7 out]
            n1359 = Greater Or Equal?(x=w1771, y=5.0) -> (x >= y?=w1770:bool)
          }
        }
        n1360 = feedback-in #28(w1660) -> ()
        n1361 = case shown="True" w1653 {
          tunnel: w1654 -> [_ w1762]
          tunnel: [TRUE FALSE] -> w1655
          tunnel: [FALSE w1763] -> w1636
          frame False {
          }
          frame True {
            n1362 = call "Elapsed Time103"("Reset"=w1762) -> ("Elapsed Time (s)"=w1764:dbl)  [unwired: 11 in, 7 out]
            n1363 = Greater Or Equal?(x=w1764, y=30.0) -> (x >= y?=w1763:bool)
          }
        }
        n1364 = feedback-in #29(w1655) -> ()
        n1365 = case shown="True" w1642 {
          tunnel: w1641 -> [_ w1755]
          tunnel: [TRUE FALSE] -> w1640
          tunnel: [FALSE w1756] -> w1635
          frame False {
          }
          frame True {
            n1366 = call "Elapsed Time104"("Reset"=w1755) -> ("Elapsed Time (s)"=w1757:dbl)  [unwired: 11 in, 7 out]
            n1367 = Greater Or Equal?(x=w1757, y=30.0) -> (x >= y?=w1756:bool)
          }
        }
        n1368 = feedback-in #30(w1640) -> ()
        n1369 = case shown="True" w1614 {
          tunnel: w1615 -> [_ w1734]
          tunnel: [TRUE FALSE] -> w1616
          tunnel: [FALSE w1735] -> _
          frame False {
          }
          frame True {
            n1370 = call "Elapsed Time107"("Reset"=w1734) -> ("Elapsed Time (s)"=w1736:dbl)  [unwired: 11 in, 7 out]
            n1371 = Greater Or Equal?(x=w1736, y=25.0) -> (x >= y?=w1735:bool)
          }
        }
        n1372 = feedback-in #31(w1616) -> ()
        n1373 = case shown="True" w1623 {
          tunnel: w1622 -> [_ w1727]
          tunnel: [TRUE FALSE] -> w1621
          tunnel: [FALSE w1728] -> _
          frame False {
          }
          frame True {
            n1374 = call "Elapsed Time108"("Reset"=w1727) -> ("Elapsed Time (s)"=w1729:dbl)  [unwired: 11 in, 7 out]
            n1375 = Greater Or Equal?(x=w1729, y=25.0) -> (x >= y?=w1728:bool)
          }
        }
        n1376 = feedback-in #32(w1621) -> ()
        n1377 = case shown="True" w1603 {
          tunnel: w1602 -> [_ w1706]
          tunnel: [TRUE FALSE] -> w1601
          tunnel: [FALSE w1707] -> w1598
          frame False {
          }
          frame True {
            n1378 = call "Elapsed Time111"("Reset"=w1706) -> ("Elapsed Time (s)"=w1708:dbl)  [unwired: 11 in, 7 out]
            n1379 = Greater Or Equal?(x=w1708, y=10.0) -> (x >= y?=w1707:bool)
          }
        }
        n1380 = feedback-in #33(w1601) -> ()
        n1381 = case shown="True" w1582 {
          tunnel: w1583 -> [_ w1685]
          tunnel: [TRUE FALSE] -> w1584
          tunnel: [FALSE w1686] -> w1587
          frame False {
          }
          frame True {
            n1382 = call "Elapsed Time113"("Reset"=w1685) -> ("Elapsed Time (s)"=w1687:dbl)  [unwired: 11 in, 7 out]
            n1383 = Greater Or Equal?(x=w1687, y=10.0) -> (x >= y?=w1686:bool)
          }
        }
        n1384 = feedback-in #34(w1584) -> ()
        n1385 = case shown="True" w1593 {
          tunnel: w1594 -> [_ w1699]
          tunnel: [TRUE FALSE] -> w1595
          tunnel: [FALSE w1700] -> _
          frame False {
          }
          frame True {
            n1386 = call "Elapsed Time112"("Reset"=w1699) -> ("Elapsed Time (s)"=w1701:dbl)  [unwired: 11 in, 7 out]
            n1387 = Greater Or Equal?(x=w1701, y=5.0) -> (x >= y?=w1700:bool)
          }
        }
        n1388 = feedback-in #35(w1595) -> ()
        n1389 = local write "ch2_pl_vbv_fail"(w1646) -> ()
        n1390 = local write "ch2_sov_fail"(w1634) -> ()
        n1391 = Or(x=w1636, y=w1635) -> (x .or. y?=w1637:bool)
        n1392 = local write "ch2_gv_bp_left_fail"(w1598) -> ()
        n1393 = local write "ch2_gv_bp_left_fail"(w1587) -> ()
        n1394 = local write "ch2_3_trns_gv_fail"(w1637) -> ()
      }
      frame #3 {
        n1395 = local read "CH3_SRV1_Piston_Back_DO"() -> (w1854:bool)
        n1396 = local read "CH3_SRV1_Piston_Back_DI"() -> (w1855:bool)
        n1397 = local read "CH3_SRV1_Piston_For_DO"() -> (w1837:bool)
        n1398 = local read "CH3_SRV1_Piston_For_DI"() -> (w1836:bool)
        n1399 = local read "CH3_CH_VBV_DO"() -> (w1896:bool)
        n1400 = local read "CH3_CH_VBV_DI"() -> (w1895:bool)
        n1401 = local read "CH3_SRV_Start_Stop_DI"() -> (w1815:bool)
        n1402 = local read "CH3_MP_DO"() -> (w1906:bool)
        n1403 = local read "CH3_MP_DI"() -> (w1905:bool)
        n1404 = local read "CH3_TP_BV_DO"() -> (w1903:bool)
        n1405 = local read "CH3_TP_BV_DI"() -> (w1904:bool)
        n1406 = local read "CH3_BG_BV_DO"() -> (w1893:bool)
        n1407 = local read "CH3_BG_BV_DI"() -> (w1894:bool)
        n1408 = local read "CH3_M3_D3_DO"() -> (w1816:bool)
        n1409 = local read "CH3_Cst_Fix_Down_DI"() -> (w1856:bool)
        n1410 = local read "CH3_WFC_DO"() -> (w1834:bool)
        n1411 = local read "CH3_WFC_DI"() -> (w1835:bool)
        n1412 = local read "CH3_Cst_Fix_DO"() -> (w1857:bool)
        n1413 = feedback #36() -> (w1891:bool)  [unwired: 1 in]
        n1414 = Exclusive Or(1:w1894, 2:w1893) -> (0:w1890:bool)
        n1415 = feedback #37() -> (w1898:bool)  [unwired: 1 in]
        n1416 = Exclusive Or(1:w1895, 2:w1896) -> (0:w1899:bool)
        n1417 = feedback #38() -> (w1908:bool)  [unwired: 1 in]
        n1418 = Exclusive Or(1:w1905, 2:w1906) -> (0:w1909:bool)
        n1419 = feedback #39() -> (w1901:bool)  [unwired: 1 in]
        n1420 = Exclusive Or(1:w1904, 2:w1903) -> (0:w1900:bool)
        n1421 = case shown="True" w1890 {
          tunnel: w1891 -> [_ w2017]
          tunnel: [TRUE FALSE] -> w1892
          tunnel: [FALSE w2018] -> w1870
          frame False {
          }
          frame True {
            n1422 = call "Elapsed Time116"("Reset"=w2017) -> ("Elapsed Time (s)"=w2019:dbl)  [unwired: 11 in, 7 out]
            n1423 = Greater Or Equal?(x=w2019, y=5.0) -> (x >= y?=w2018:bool)
          }
        }
        n1424 = feedback-in #36(w1892) -> ()
        n1425 = case shown="True" w1899 {
          tunnel: w1898 -> [_ w2010]
          tunnel: [TRUE FALSE] -> w1897
          tunnel: [FALSE w2011] -> w1872
          frame False {
          }
          frame True {
            n1426 = call "Elapsed Time117"("Reset"=w2010) -> ("Elapsed Time (s)"=w2012:dbl)  [unwired: 11 in, 7 out]
            n1427 = Greater Or Equal?(x=w2012, y=5.0) -> (x >= y?=w2011:bool)
          }
        }
        n1428 = feedback-in #37(w1897) -> ()
        n1429 = feedback #40() -> (w1832:bool)  [unwired: 1 in]
        n1430 = Exclusive Or(1:w1835, 2:w1834) -> (0:w1831:bool)
        n1431 = feedback #41() -> (w1818:bool)  [unwired: 1 in]
        n1432 = Exclusive Or(1:w1815, 2:w1816) -> (0:w1819:bool)
        n1433 = case shown="True" w1909 {
          tunnel: w1908 -> [_ w2031]
          tunnel: [TRUE FALSE] -> w1907
          tunnel: [FALSE w2032] -> w1874
          frame False {
          }
          frame True {
            n1434 = call "Elapsed Time114"("Reset"=w2031) -> ("Elapsed Time (s)"=w2033:dbl)  [unwired: 11 in, 7 out]
            n1435 = Greater Or Equal?(x=w2033, y=5.0) -> (x >= y?=w2032:bool)
          }
        }
        n1436 = feedback-in #38(w1907) -> ()
        n1437 = case shown="True" w1900 {
          tunnel: w1901 -> [_ w2024]
          tunnel: [TRUE FALSE] -> w1902
          tunnel: [FALSE w2025] -> w1871
          frame False {
          }
          frame True {
            n1438 = call "Elapsed Time115"("Reset"=w2024) -> ("Elapsed Time (s)"=w2026:dbl)  [unwired: 11 in, 7 out]
            n1439 = Greater Or Equal?(x=w2026, y=5.0) -> (x >= y?=w2025:bool)
          }
        }
        n1440 = feedback-in #39(w1902) -> ()
        n1441 = feedback #42() -> (w1859:bool)  [unwired: 1 in]
        n1442 = Exclusive Or(1:w1856, 2:w1857) -> (0:w1860:bool)
        n1443 = feedback #43() -> (w1852:bool)  [unwired: 1 in]
        n1444 = Exclusive Or(1:w1855, 2:w1854) -> (0:w1851:bool)
        n1445 = feedback #44() -> (w1839:bool)  [unwired: 1 in]
        n1446 = Exclusive Or(1:w1836, 2:w1837) -> (0:w1840:bool)
        n1447 = case shown="True" w1831 {
          tunnel: w1832 -> [_ w1940]
          tunnel: [TRUE FALSE] -> w1833
          tunnel: [FALSE w1941] -> _
          frame False {
          }
          frame True {
            n1448 = call "Elapsed Time127"("Reset"=w1940) -> ("Elapsed Time (s)"=w1942:dbl)  [unwired: 11 in, 7 out]
            n1449 = Greater Or Equal?(x=w1942, y=5.0) -> (x >= y?=w1941:bool)
          }
        }
        n1450 = feedback-in #40(w1833) -> ()
        n1451 = case shown="True" w1819 {
          tunnel: w1818 -> [_ w1919]
          tunnel: [TRUE FALSE] -> w1817
          tunnel: [FALSE w1920] -> _
          frame False {
          }
          frame True {
            n1452 = call "Elapsed Time130"("Reset"=w1919) -> ("Elapsed Time (s)"=w1921:dbl)  [unwired: 11 in, 7 out]
            n1453 = Greater Or Equal?(x=w1921, y=5.0) -> (x >= y?=w1920:bool)
          }
        }
        n1454 = feedback-in #41(w1817) -> ()
        n1455 = case shown="True" w1860 {
          tunnel: w1859 -> [_ w1975]
          tunnel: [TRUE FALSE] -> w1858
          tunnel: [FALSE w1976] -> _
          frame False {
          }
          frame True {
            n1456 = call "Elapsed Time122"("Reset"=w1975) -> ("Elapsed Time (s)"=w1977:dbl)  [unwired: 11 in, 7 out]
            n1457 = Greater Or Equal?(x=w1977, y=20.0) -> (x >= y?=w1976:bool)
          }
        }
        n1458 = feedback-in #42(w1858) -> ()
        n1459 = case shown="True" w1851 {
          tunnel: w1852 -> [_ w1968]
          tunnel: [TRUE FALSE] -> w1853
          tunnel: [FALSE w1969] -> _
          frame False {
          }
          frame True {
            n1460 = call "Elapsed Time123"("Reset"=w1968) -> ("Elapsed Time (s)"=w1970:dbl)  [unwired: 11 in, 7 out]
            n1461 = Greater Or Equal?(x=w1970, y=25.0) -> (x >= y?=w1969:bool)
          }
        }
        n1462 = feedback-in #43(w1853) -> ()
        n1463 = case shown="True" w1840 {
          tunnel: w1839 -> [_ w1947]
          tunnel: [TRUE FALSE] -> w1838
          tunnel: [FALSE w1948] -> _
          frame False {
          }
          frame True {
            n1464 = call "Elapsed Time126"("Reset"=w1947) -> ("Elapsed Time (s)"=w1949:dbl)  [unwired: 11 in, 7 out]
            n1465 = Greater Or Equal?(x=w1949, y=25.0) -> (x >= y?=w1948:bool)
          }
        }
        n1466 = feedback-in #44(w1838) -> ()
        n1467 = local write "ch3_ch_vbv_fail"(w1872) -> ()
        n1468 = local write "ch3_mp_fail"(w1874) -> ()
        n1469 = local write "ch3_tp_bv_fail"(w1871) -> ()
        n1470 = local write "ch3_bg_bv_fail"(w1870) -> ()
        n1471 = local read "CH3_Trns_GV_Open_DO"() -> (w1883:bool)
        n1472 = local read "CH3_Trns_GV_Close_DO"() -> (w1866:bool)
        n1473 = local read "CH3_Trns_BP_Right_DO"() -> (w1812:bool)
        n1474 = local read "CH3_Trns_BP_Right_DI"() -> (w1813:bool)
        n1475 = local read "CH3_Trns_Gv_Open_DI"() -> (w1884:bool)
        n1476 = local read "CH3_Trns_Gv_Close_DI"() -> (w1865:bool)
        n1477 = local read "CH3_Trns_BP_Left_DO"() -> (w1827:bool)
        n1478 = local read "CH3_Trns_BP_Left_DI"() -> (w1826:bool)
        n1479 = local read "CH3_TGV_Control_DO"() -> (w1823:bool)
        n1480 = local read "CH3_TGV_Control_DI"() -> (w1824:bool)
        n1481 = local read "CH3_PetCool_Up_DO"() -> (w1847:bool)
        n1482 = local read "CH3_PetCool_Up_DI"() -> (w1846:bool)
        n1483 = local read "CH3_PetCool_Down_DO"() -> (w1844:bool)
        n1484 = local read "CH3_PetCool_Down_DI"() -> (w1845:bool)
        n1485 = local read "CH3_PL_VBV_DO"() -> (w1878:bool)
        n1486 = local read "CH3_PL_VBV_DI"() -> (w1879:bool)
        n1487 = local read "CH3_SoV_Ar_DO"() -> (w1886:bool)
        n1488 = local read "CH3_SoV_Ar_DI"() -> (w1885:bool)
        n1489 = feedback #45() -> (w1876:bool)  [unwired: 1 in]
        n1490 = Exclusive Or(1:w1879, 2:w1878) -> (0:w1875:bool)
        n1491 = feedback #46() -> (w1888:bool)  [unwired: 1 in]
        n1492 = Exclusive Or(1:w1885, 2:w1886) -> (0:w1889:bool)
        n1493 = feedback #47() -> (w1881:bool)  [unwired: 1 in]
        n1494 = Exclusive Or(1:w1884, 2:w1883) -> (0:w1880:bool)
        n1495 = feedback #48() -> (w1868:bool)  [unwired: 1 in]
        n1496 = Exclusive Or(1:w1865, 2:w1866) -> (0:w1869:bool)
        n1497 = feedback #49() -> (w1842:bool)  [unwired: 1 in]
        n1498 = Exclusive Or(1:w1845, 2:w1844) -> (0:w1841:bool)
        n1499 = feedback #50() -> (w1849:bool)  [unwired: 1 in]
        n1500 = Exclusive Or(1:w1846, 2:w1847) -> (0:w1850:bool)
        n1501 = feedback #51() -> (w1829:bool)  [unwired: 1 in]
        n1502 = Exclusive Or(1:w1826, 2:w1827) -> (0:w1830:bool)
        n1503 = feedback #52() -> (w1810:bool)  [unwired: 1 in]
        n1504 = Exclusive Or(1:w1813, 2:w1812) -> (0:w1809:bool)
        n1505 = feedback #53() -> (w1821:bool)  [unwired: 1 in]
        n1506 = Exclusive Or(1:w1824, 2:w1823) -> (0:w1820:bool)
        n1507 = case shown="True" w1875 {
          tunnel: w1876 -> [_ w2003]
          tunnel: [TRUE FALSE] -> w1877
          tunnel: [FALSE w2004] -> w1873
          frame False {
          }
          frame True {
            n1508 = call "Elapsed Time118"("Reset"=w2003) -> ("Elapsed Time (s)"=w2005:dbl)  [unwired: 11 in, 7 out]
            n1509 = Greater Or Equal?(x=w2005, y=5.0) -> (x >= y?=w2004:bool)
          }
        }
        n1510 = feedback-in #45(w1877) -> ()
        n1511 = case shown="True" w1889 {
          tunnel: w1888 -> [_ w1996]
          tunnel: [TRUE FALSE] -> w1887
          tunnel: [FALSE w1997] -> w1861
          frame False {
          }
          frame True {
            n1512 = call "Elapsed Time119"("Reset"=w1996) -> ("Elapsed Time (s)"=w1998:dbl)  [unwired: 11 in, 7 out]
            n1513 = Greater Or Equal?(x=w1998, y=5.0) -> (x >= y?=w1997:bool)
          }
        }
        n1514 = feedback-in #46(w1887) -> ()
        n1515 = case shown="True" w1880 {
          tunnel: w1881 -> [_ w1989]
          tunnel: [TRUE FALSE] -> w1882
          tunnel: [FALSE w1990] -> w1863
          frame False {
          }
          frame True {
            n1516 = call "Elapsed Time120"("Reset"=w1989) -> ("Elapsed Time (s)"=w1991:dbl)  [unwired: 11 in, 7 out]
            n1517 = Greater Or Equal?(x=w1991, y=30.0) -> (x >= y?=w1990:bool)
          }
        }
        n1518 = feedback-in #47(w1882) -> ()
        n1519 = case shown="True" w1869 {
          tunnel: w1868 -> [_ w1982]
          tunnel: [TRUE FALSE] -> w1867
          tunnel: [FALSE w1983] -> w1862
          frame False {
          }
          frame True {
            n1520 = call "Elapsed Time121"("Reset"=w1982) -> ("Elapsed Time (s)"=w1984:dbl)  [unwired: 11 in, 7 out]
            n1521 = Greater Or Equal?(x=w1984, y=30.0) -> (x >= y?=w1983:bool)
          }
        }
        n1522 = feedback-in #48(w1867) -> ()
        n1523 = case shown="True" w1841 {
          tunnel: w1842 -> [_ w1961]
          tunnel: [TRUE FALSE] -> w1843
          tunnel: [FALSE w1962] -> _
          frame False {
          }
          frame True {
            n1524 = call "Elapsed Time124"("Reset"=w1961) -> ("Elapsed Time (s)"=w1963:dbl)  [unwired: 11 in, 7 out]
            n1525 = Greater Or Equal?(x=w1963, y=25.0) -> (x >= y?=w1962:bool)
          }
        }
        n1526 = feedback-in #49(w1843) -> ()
        n1527 = case shown="True" w1850 {
          tunnel: w1849 -> [_ w1954]
          tunnel: [TRUE FALSE] -> w1848
          tunnel: [FALSE w1955] -> _
          frame False {
          }
          frame True {
            n1528 = call "Elapsed Time125"("Reset"=w1954) -> ("Elapsed Time (s)"=w1956:dbl)  [unwired: 11 in, 7 out]
            n1529 = Greater Or Equal?(x=w1956, y=25.0) -> (x >= y?=w1955:bool)
          }
        }
        n1530 = feedback-in #50(w1848) -> ()
        n1531 = case shown="True" w1830 {
          tunnel: w1829 -> [_ w1933]
          tunnel: [TRUE FALSE] -> w1828
          tunnel: [FALSE w1934] -> w1825
          frame False {
          }
          frame True {
            n1532 = call "Elapsed Time128"("Reset"=w1933) -> ("Elapsed Time (s)"=w1935:dbl)  [unwired: 11 in, 7 out]
            n1533 = Greater Or Equal?(x=w1935, y=10.0) -> (x >= y?=w1934:bool)
          }
        }
        n1534 = feedback-in #51(w1828) -> ()
        n1535 = case shown="True" w1809 {
          tunnel: w1810 -> [_ w1912]
          tunnel: [TRUE FALSE] -> w1811
          tunnel: [FALSE w1913] -> w1814
          frame False {
          }
          frame True {
            n1536 = call "Elapsed Time131"("Reset"=w1912) -> ("Elapsed Time (s)"=w1914:dbl)  [unwired: 11 in, 7 out]
            n1537 = Greater Or Equal?(x=w1914, y=10.0) -> (x >= y?=w1913:bool)
          }
        }
        n1538 = feedback-in #52(w1811) -> ()
        n1539 = case shown="True" w1820 {
          tunnel: w1821 -> [_ w1926]
          tunnel: [TRUE FALSE] -> w1822
          tunnel: [FALSE w1927] -> _
          frame False {
          }
          frame True {
            n1540 = call "Elapsed Time129"("Reset"=w1926) -> ("Elapsed Time (s)"=w1928:dbl)  [unwired: 11 in, 7 out]
            n1541 = Greater Or Equal?(x=w1928, y=5.0) -> (x >= y?=w1927:bool)
          }
        }
        n1542 = feedback-in #53(w1822) -> ()
        n1543 = local write "ch3_gv_bp_right_fail"(w1814) -> ()
        n1544 = local write "ch3_pl_vbv_fail"(w1873) -> ()
        n1545 = local write "ch3_sov_fail"(w1861) -> ()
        n1546 = Or(x=w1863, y=w1862) -> (x .or. y?=w1864:bool)
        n1547 = local write "ch3_gv_bp_left_fail"(w1825) -> ()
        n1548 = local write "ch3_4_trns_gv_fail"(w1864) -> ()
      }
      frame #4 {
        n1549 = local read "CH4_TGV_Control_DO"() -> (w2050:bool)
        n1550 = local read "CH4_TGV_Control_DI"() -> (w2051:bool)
        n1551 = local read "CH4_SRV1_Piston_For_DI"() -> (w2042:bool)
        n1552 = local read "CH4_CH_VBV_DO"() -> (w2104:bool)
        n1553 = local read "CH4_CH_VBV_DI"() -> (w2103:bool)
        n1554 = local read "CH4_MP_DO"() -> (w2114:bool)
        n1555 = local read "CH4_MP_DI"() -> (w2113:bool)
        n1556 = local read "CH4_TP_BV_DO"() -> (w2111:bool)
        n1557 = local read "CH4_TP_BV_DI"() -> (w2112:bool)
        n1558 = local read "CH4_BG_BV_DO"() -> (w2101:bool)
        n1559 = local read "CH4_BG_BV_DI"() -> (w2102:bool)
        n1560 = local read "CH4_WFC_DO"() -> (w2055:bool)
        n1561 = local read "CH4_WFC_DI"() -> (w2056:bool)